vi "Main.vi"() -> ()   [LabVIEW 2015] (continued)
                n1016 = local read "G_max"() -> (w1896:dbl)
                n1017 = local read "G_min"() -> (w1895:dbl)
                n1018 = local read "S_max"() -> (w1894:dbl)
                n1019 = local read "S_min"() -> (w1893:dbl)
                n1020 = Square(x=w1924) -> (x^2=w1922:dbl)
                n1021 = Square(x=w1923) -> (x^2=w1921:dbl)
                n1022 = Add(x=w1922, y=w1921) -> (x+y=w1920:dbl)
                n1023 = Square Root(x=w1920) -> (sqrt(x)=w1919:dbl)
                n1024 = call "DrawROICircle.vi"("old picture"=w1917, "ROI?"=w1912, "Radius (G/S)"=w1911, "Center (G/S)"=w1910, "PicSize"=w1916, "Color"=w1909, "G_max"=w1896, "S_max"=w1894, "G_min"=w1895, "S_min"=w1893) -> ("new picture"=w1915:picture)  [unwired: 9 in]
                n1025 = call "DrawROICircle.vi"("old picture"=w1915, "ROI?"=w1907, "Radius (G/S)"=w1908, "Center (G/S)"=w1898, "PicSize"=w1916, "Color"=w1906, "G_max"=w1896, "S_max"=w1894, "G_min"=w1895, "S_min"=w1893) -> ("new picture"=w1903:picture)  [unwired: 9 in]
                n1026 = call "DrawROICircle.vi"("old picture"=w1903, "ROI?"=w1892, "Radius (G/S)"=w1905, "Center (G/S)"=w1897, "PicSize"=w1916, "Color"=w1904, "G_max"=w1896, "S_max"=w1894, "G_min"=w1895, "S_min"=w1893) -> ("new picture"=w1914:picture)  [unwired: 9 in]
                n1027 = call "DrawROICircle.vi"("old picture"=w1914, "ROI?"=w1902, "Radius (G/S)"=w1901, "Center (G/S)"=w1900, "PicSize"=w1916, "Color"=w1899, "G_max"=w1896, "S_max"=w1894, "G_min"=w1895, "S_min"=w1893) -> ("new picture"=w1913:picture)  [unwired: 9 in]
                n1028 = case shown="\"ROI4\"" w1918 {
                  tunnel: w1919 -> [_ w1928 w1929 w1930 w1931]
                  frame "None" {
                  }
                  frame "ROI1" {
                    "Radius1" <- w1928
                  }
                  frame "ROI2" {
                    "Radius2" <- w1929
                  }
                  frame "ROI3" {
                    "Radius3" <- w1930
                  }
                  frame "ROI4" {
                    "Radius4" <- w1931
                  }
                }
              }
            }
          }
        }
        n1029 = property on="Phasor Plot" class="IntGraph (strict)"(error in=w1816, "PlotImages.Front"=w1817) -> (error out=w1822:errorcluster)  [unwired: 1 in, 1 out]
      }
      event "Phasor Plot": Mouse Up; "ROI1?", "ROI2?", "ROI3?", "ROI4?", "Phasor\nOverlap?", "Refresh Overlap": Value Change {
        n1030 = event-data() -> ()  [unwired: 1 in, 1 out]
        n1031 = local read "ROI Drawing"() -> (w1976:bool)
        n1032 = local read "ROI Select"() -> (w1977:enum16{"None", "ROI1", "ROI2", "ROI3", "ROI4"})
        n1033 = case shown="True" w1976 {
          tunnel: w1977 -> [_ w2002]
          tunnel: w1969 -> [w1999 w2000]
          tunnel: [w1999 w2000] -> w1968
          frame False {
          }
          frame True {
            n1034 = case shown="\"ROI1\"" w2002 {
              frame "None" {
              }
              frame "ROI1" {
                n1035 = local read "Radius1"() -> (w2007:dbl)
                n1036 = Greater Than 0?(x=w2007) -> (x > 0?=w2006:bool)
                n1037 = Select(t=TRUE ("ROI Drawing"), s=w2006, f=FALSE ("ROI Drawing")) -> (s? t:f=w2005:bool)
                n1038 = local write "ROI1?"(w2005) -> ()
              }
              frame "ROI2" {
                n1039 = local read "Radius2"() -> (w2009:dbl)
                n1040 = Greater Than 0?(x=w2009) -> (x > 0?=w2012:bool)
                n1041 = Select(t=TRUE ("ROI Drawing"), s=w2012, f=FALSE ("ROI Drawing")) -> (s? t:f=w2008:bool)
                n1042 = local write "ROI2?"(w2008) -> ()
              }
              frame "ROI3" {
                n1043 = local read "Radius3"() -> (w2015:dbl)
                n1044 = Greater Than 0?(x=w2015) -> (x > 0?=w2016:bool)
                n1045 = Select(t=TRUE ("ROI Drawing"), s=w2016, f=FALSE ("ROI Drawing")) -> (s? t:f=w2014:bool)
                n1046 = local write "ROI3?"(w2014) -> ()
              }
              frame "ROI4" {
                n1047 = local read "Radius4"() -> (w2019:dbl)
                n1048 = Greater Than 0?(x=w2019) -> (x > 0?=w2022:bool)
                n1049 = Select(t=TRUE ("ROI Drawing"), s=w2022, f=FALSE ("ROI Drawing")) -> (s? t:f=w2018:bool)
                n1050 = local write "ROI4?"(w2018) -> ()
              }
            }
            n1051 = local write "ROI Drawing"(FALSE ("ROI Drawing")) -> ()
          }
        }
        n1052 = local read "Radius4"() -> (w1964:dbl)
        n1053 = local read "Center4"() -> (w1961:cluster{dbl, dbl})
        n1054 = local read "Radius2"() -> (w1966:dbl)
        n1055 = local read "Center2"() -> (w1962:cluster{dbl, dbl})
        n1056 = local read "Radius3"() -> (w1965:dbl)
        n1057 = local read "Center3"() -> (w1952:cluster{dbl, dbl})
        n1058 = local read "Radius1"() -> (w1967:dbl)
        n1059 = local read "Center1"() -> (w1963:cluster{dbl, dbl})
        n1060 = local read "PicSize"() -> (w1972:u32)
        n1061 = local read "Color4"() -> (w1957:u32)
        n1062 = local read "Color2"() -> (w1959:u32)
        n1063 = local read "Color3"() -> (w1958:u32)
        n1064 = local read "Color1"() -> (w1960:u32)
        n1065 = local read "ROI4?"() -> (w1942:bool)
        n1066 = local read "ROI3?"() -> (w1943:bool)
        n1067 = local read "ROI1?"() -> (w1945:bool)
        n1068 = local read "ROI2?"() -> (w1944:bool)
        n1069 = Build Array(w1945, w1944, w1943, w1942) -> (w1941:bool[])
        n1070 = Build Array(w1967, w1966, w1965, w1964) -> (w1940:dbl[])
        n1071 = Build Array(w1963, w1962, w1952, w1961) -> (w1939:cluster{dbl, dbl}[])
        n1072 = local read "G_max"() -> (w1951:dbl)
        n1073 = local read "G_min"() -> (w1950:dbl)
        n1074 = local read "S_max"() -> (w1949:dbl)
        n1075 = Build Array(w1960, w1959, w1958, w1957) -> (w1938:u32[])
        n1076 = local read "S_min"() -> (w1948:dbl)
        n1077 = call "Empty Picture"() -> ("empty picture"=w1970:picture)
        n1078 = call "DrawROICircle.vi"("old picture"=w1970, "ROI?"=w1945, "Radius (G/S)"=w1967, "Center (G/S)"=w1963, "PicSize"=w1972, "Color"=w1960, "G_max"=w1951, "S_max"=w1949, "G_min"=w1950, "S_min"=w1948) -> ("new picture"=w1975:picture)  [unwired: 9 in]
        n1079 = call "DrawROICircle.vi"("old picture"=w1975, "ROI?"=w1944, "Radius (G/S)"=w1966, "Center (G/S)"=w1962, "PicSize"=w1972, "Color"=w1959, "G_max"=w1951, "S_max"=w1949, "G_min"=w1950, "S_min"=w1948) -> ("new picture"=w1973:picture)  [unwired: 9 in]
        n1080 = call "DrawROICircle.vi"("old picture"=w1973, "ROI?"=w1943, "Radius (G/S)"=w1965, "Center (G/S)"=w1952, "PicSize"=w1972, "Color"=w1958, "G_max"=w1951, "S_max"=w1949, "G_min"=w1950, "S_min"=w1948) -> ("new picture"=w1974:picture)  [unwired: 9 in]
        n1081 = call "DrawROICircle.vi"("old picture"=w1974, "ROI?"=w1942, "Radius (G/S)"=w1964, "Center (G/S)"=w1961, "PicSize"=w1972, "Color"=w1957, "G_max"=w1951, "S_max"=w1949, "G_min"=w1950, "S_min"=w1948) -> ("new picture"=w1971:picture)  [unwired: 9 in]
        n1082 = local read "Auto Scale?"() -> (w1936:bool)
        n1083 = local read "Max Intensity"() -> (w1935:dbl)
        n1084 = local read "Min Intensity"() -> (w1934:dbl)
        n1085 = control-ref of="Image with Phasors"() -> (w1954:refnum<vi>)
        n1086 = property on="Phasor Plot" class="IntGraph (strict)"(error in=w1968, "PlotImages.Front"=w1971) -> (error out=w1947:errorcluster)  [unwired: 1 in, 1 out]
        n1087 = Bundle(w1941, w1940, w1939, w1938) -> (→"ROI Cluster":T9)  [unwired: 1 in]
        n1088 = local read "V_DC"() -> (w1953:dbl[][])
        n1089 = case shown="True" "Phasor\nOverlap?" {
          tunnel: w1941 -> [_ w1996]
          tunnel: w1940 -> [_ w1995]
          tunnel: w1939 -> [_ w1994]
          tunnel: w1938 -> [_ w1993]
          tunnel: [w1986 w1992] -> w1955
          tunnel: w1954 -> [w1985 w1991]
          tunnel: w1936 -> [w1983 w1990]
          tunnel: w1935 -> [w1982 w1989]
          tunnel: w1934 -> [w1981 w1988]
          tunnel: w1953 -> [w1984 w1987]
          frame False {
            n1090 = call "Array2GrayPic.vi"("Pic Reference"=w1985, "Threshold (min)"=w1981, "Threshold (max)"=w1982, "Auto Scale?"=w1983, "Intensity"=w1984) -> ("Gray Picture"=w1986:picture)  [unwired: 6 in]
          }
          frame True {
            n1091 = local read "G Data"() -> (w1998:dbl[][])
            n1092 = local read "S Data"() -> (w1997:dbl[][])
            n1093 = call "PhasorROI2IMG.vi"("Intensity"=w1987, "Auto Scale?"=w1990, "Threshold (max)"=w1989, "Threshold (min)"=w1988, "G Data"=w1998, "S Data"=w1997, "Pic Reference"=w1991, "ROI? array"=w1996, "Radius array"=w1995, "Center array"=w1994, "Color array"=w1993) -> ("new picture"=w1992:picture)  [unwired: 8 in]
          }
        }
        n1094 = flat-sequence {
          tunnel: [w1980] -> w1946
          tunnel: w1947 -> [w1980]
          frame #0 {
            n1095 = local write "Refresh Overlap"(FALSE ("Fast Scan")) -> ()
          }
        }
        n1096 = local write "Image with Phasors"(w1955) -> ()
      }
      event "Phasor Grids", "G_max", "G_min", "S_max", "S_min", "Phasor Colormap", "Update Phasor": Value Change {
        n1097 = event-data() -> ()  [unwired: 1 in, 1 out]
        n1098 = local read "Phasor Colormap"() -> (w2028:T8)
        n1099 = local read "Max Intensity"() -> (w2026:dbl)
        n1100 = local read "Min Intensity"() -> (w2025:dbl)
        n1101 = local read "Auto Scale?"() -> (w2027:bool)
        n1102 = control-ref of="Phasor Plot"() -> (w2029:refnum<vi>)
        n1103 = local read "Phasor Grids"() -> (w2030:i32)
        n1104 = local read "V_DC"() -> (w2033:dbl[][])
        n1105 = control-ref of="Image with Phasors"() -> (w2042:refnum<vi>)
        n1106 = local read "G Data"() -> (w2032:dbl[][])
        n1107 = local read "S Data"() -> (w2031:dbl[][])
        n1108 = local read "G_max"() -> (w2037:dbl)
        n1109 = local read "G_min"() -> (w2036:dbl)
        n1110 = local read "S_max"() -> (w2035:dbl)
        n1111 = local read "S_min"() -> (w2034:dbl)
        n1112 = call "Array2GrayPic.vi"("Pic Reference"=w2042, "Threshold (min)"=w2025, "Threshold (max)"=w2026, "Auto Scale?"=w2027, "Intensity"=w2033) -> ("Gray Picture"=w2041:picture)  [unwired: 6 in]
        n1113 = call "DrawPhasorPlot.vi"("Intensity"=w2033, "G Data"=w2032, "S Data"=w2031, "Threshold (max)"=w2026, "Threshold (min)"=w2025, "error in"=w2040, "G_max"=w2037, "Auto Scale?"=w2027, "G_min"=w2036, "Phasor Grids"=w2030, "S_max"=w2035, "Reference"=w2029, "S_min"=w2034, "Phasor Colormap"=w2028) -> ("Phasor Plot"=w2038:dbl[][], "error out"=w2039:errorcluster)  [unwired: 4 in]
        n1114 = local write "Image with Phasors"(w2041) -> ()
        n1115 = local write "Phasor Plot"(w2038) -> ()
      }
      event "Load P1": Value Change {
        n1116 = event-data() -> ()  [unwired: 1 in, 1 out]
        n1117 = local read "Measurement Parameters"() -> (w2063:T4)
        n1118 = property on="Composite q1,1" class="Pict"(error in=w2060) -> (error out=w2059:errorcluster, "Draw Area Size"=w2064:T16)  [unwired: 1 in, 1 out]
        n1119 = local read "V_DC"() -> (→"DC,1":dbl[][])
        n1120 = local read "V_IF (pi)"() -> (w2085:dbl[][])
        n1121 = local read "V_IF (0)"() -> (w2084:dbl[][])
        n1122 = local read "V_IF (0.5pi)"() -> (w2083:dbl[][])
        n1123 = local read "V_IF (1.5pi)"() -> (w2082:dbl[][])
        n1124 = Unbundle By Name(w2063) -> ("Pixel Size"=w2062:dbl)
        n1125 = Unbundle By Name(w2064) -> ("Width"=w2065:u32)
        n1126 = To Single Precision Float(number=w2065) -> (single precision float=w2067:sgl)
        n1127 = To Single Precision Float(number=w2062) -> (single precision float=w2066:sgl)
        n1128 = Divide(x=w2067, y=w2066) -> (x/y=w2061:sgl)
        n1129 = Subtract(x=w2085, y=w2084) -> (x-y=w2077:dbl[][])
        n1130 = Subtract(x=w2083, y=w2082) -> (x-y=w2078:dbl[][])
        n1131 = property on="Composite q1,1" class="Pict"(error in=w2059, "ZoomFactor"=w2061) -> (error out=w2055:errorcluster)  [unwired: 1 in, 1 out]
        n1132 = local read "tau_max (s)"() -> (w2057:dbl)
        n1133 = local read "tau_min (s)"() -> (w2056:dbl)
        n1134 = Square(x=w2077) -> (x^2=w2081:dbl[][])
        n1135 = Square(x=w2078) -> (x^2=w2080:dbl[][])
        n1136 = Divide(x=w2077, y=w2078) -> (x/y=w2076:dbl[][])
        n1137 = Add(x=w2081, y=w2080) -> (x+y=w2079:dbl[][])
        n1138 = Inverse Tangent(1:w2076) -> (0:w2073:dbl[][])
        "Angle q1,1" <- w2073
        n1139 = property on="Lifetime q1,1" class="IntGraph (strict)"(error in=w2055, "ZScale.Minimum"=w2056) -> (error out=w2054:errorcluster)  [unwired: 1 in, 1 out]
        n1140 = Square Root(x=w2079) -> (sqrt(x)=w2052:dbl[][])
        "Mag q1,1" <- w2052
        n1141 = Tangent(1:w2073) -> (0:w2072:dbl[][])
        n1142 = Multiply(x=80000000.0, y=6.283185307179586) -> (x*y=w2071:dbl)
        n1143 = local read "Custom Mag?"() -> (w2053:bool)
        n1144 = Divide(x=w2072, y=w2071) -> (x/y=w2070:dbl[][])
        n1145 = property on="Lifetime q1,1" class="IntGraph (strict)"(error in=w2054, "ZScale.Maximum"=w2057) -> (error out=w2051:errorcluster)  [unwired: 1 in, 1 out]
        n1146 = Negate(x=w2070) -> (-x=w2068:dbl[][])
        "Lifetime q1,1" <- w2068
        n1147 = case shown="True" w2053 {
          tunnel: w2052 -> [w2089 _]
          tunnel: [w2088 "q1,1max"] -> w2047
          tunnel: [w2087 "q1,1min"] -> w2048
          frame False {
            n1148 = Array Max & Min(array=w2089) -> (max value=w2088:dbl, min value=w2087:dbl)  [unwired: 2 out]
          }
          frame True {
          }
        }
        n1149 = call "HSVCombIntensityLifetime.vi"("min_intensity"=w2048, "Auto Scale?"=TRUE ("External Bound Intensity Value?"), "max_intensity"=w2047, "lifetime_max (s)"=w2057, "lifetime_min (s)"=w2056, "Lifetime image"=w2068, "Intensity image"=w2052) -> ("HSV to RGB Picture"=→"Composite q1,1":picture)  [unwired: 1 in, 3 out]
        n1150 = property on="Mag q1,1" class="IntGraph (strict)"(error in=w2051, "ZScale.Minimum"=w2048) -> (error out=w2050:errorcluster)  [unwired: 1 in, 1 out]
        n1151 = property on="Mag q1,1" class="IntGraph (strict)"(error in=w2050, "ZScale.Maximum"=w2047) -> (error out=w2049:errorcluster)  [unwired: 1 in, 1 out]
      }
      event "Load P2": Value Change {
        n1152 = event-data() -> ()  [unwired: 1 in, 1 out]
        n1153 = local read "Measurement Parameters"() -> (w2111:T4)
        n1154 = property on="Composite q1,2" class="Pict"(error in=w2110) -> (error out=w2109:errorcluster, "Draw Area Size"=w2108:T16)  [unwired: 1 in, 1 out]
        n1155 = Unbundle By Name(w2111) -> ("Pixel Size"=w2112:dbl)
        n1156 = local read "V_IF (pi)"() -> (w2127:dbl[][])
        n1157 = local read "V_IF (0)"() -> (w2126:dbl[][])
        n1158 = local read "V_IF (0.5pi)"() -> (w2125:dbl[][])
        n1159 = local read "V_IF (1.5pi)"() -> (w2124:dbl[][])
        n1160 = local read "V_DC"() -> (→"DC,2":dbl[][])
        n1161 = Unbundle By Name(w2108) -> ("Width"=w2113:u32)
        n1162 = To Single Precision Float(number=w2113) -> (single precision float=w2115:sgl)
        n1163 = To Single Precision Float(number=w2112) -> (single precision float=w2114:sgl)
        n1164 = Divide(x=w2115, y=w2114) -> (x/y=w2107:sgl)
        n1165 = Subtract(x=w2127, y=w2126) -> (x-y=w2129:dbl[][])
        n1166 = Subtract(x=w2125, y=w2124) -> (x-y=w2130:dbl[][])
        n1167 = property on="Composite q1,2" class="Pict"(error in=w2109, "ZoomFactor"=w2107) -> (error out=w2102:errorcluster)  [unwired: 1 in, 1 out]
        n1168 = local read "tau_max (s)"() -> (w2105:dbl)
        n1169 = local read "tau_min (s)"() -> (w2106:dbl)
        n1170 = Square(x=w2129) -> (x^2=w2133:dbl[][])
        n1171 = Square(x=w2130) -> (x^2=w2132:dbl[][])
        n1172 = Divide(x=w2129, y=w2130) -> (x/y=w2128:dbl[][])
        n1173 = property on="Lifetime q1,2" class="IntGraph (strict)"(error in=w2102, "ZScale.Minimum"=w2106) -> (error out=w2101:errorcluster)  [unwired: 1 in, 1 out]
        n1174 = Add(x=w2133, y=w2132) -> (x+y=w2131:dbl[][])
        n1175 = Inverse Tangent(1:w2128) -> (0:w2095:dbl[][])
        "Angle q1,2" <- w2095
        n1176 = local read "Custom Mag?"() -> (w2104:bool)
        n1177 = property on="Lifetime q1,2" class="IntGraph (strict)"(error in=w2101, "ZScale.Maximum"=w2105) -> (error out=w2100:errorcluster)  [unwired: 1 in, 1 out]
        n1178 = Square Root(x=w2131) -> (sqrt(x)=w2103:dbl[][])
        "Mag q1,2" <- w2103
        n1179 = Tangent(1:w2095) -> (0:w2121:dbl[][])
        n1180 = Multiply(x=80000000.0, y=6.283185307179586) -> (x*y=w2120:dbl)
        n1181 = case shown="True" w2104 {
          tunnel: w2103 -> [w2137 _]
          tunnel: [w2136 "q1,2max"] -> w2097
          tunnel: [w2135 "q1,2min"] -> w2096
          frame False {
            n1182 = Array Max & Min(array=w2137) -> (max value=w2136:dbl, min value=w2135:dbl)  [unwired: 2 out]
          }
          frame True {
          }
        }
        n1183 = Divide(x=w2121, y=w2120) -> (x/y=w2119:dbl[][])
        n1184 = Negate(x=w2119) -> (-x=w2117:dbl[][])
        "Lifetime q1,2" <- w2117
        n1185 = call "HSVCombIntensityLifetime.vi"("min_intensity"=w2096, "Auto Scale?"=TRUE ("External Bound Intensity Value?"), "max_intensity"=w2097, "lifetime_max (s)"=w2105, "lifetime_min (s)"=w2106, "Lifetime image"=w2117, "Intensity image"=w2103) -> ("HSV to RGB Picture"=→"Composite q1,2":picture)  [unwired: 1 in, 3 out]
        n1186 = property on="Mag q1,2" class="IntGraph (strict)"(error in=w2100, "ZScale.Minimum"=w2096) -> (error out=w2099:errorcluster)  [unwired: 1 in, 1 out]
        n1187 = property on="Mag q1,2" class="IntGraph (strict)"(error in=w2099, "ZScale.Maximum"=w2097) -> (error out=w2098:errorcluster)  [unwired: 1 in, 1 out]
      }
      event "Two-Step GSOS": Value Change {
        n1188 = event-data() -> ()  [unwired: 1 in, 1 out]
        n1189 = local read "Measurement Parameters"() -> (w2162:T4)
        n1190 = property on="Composite GSOS" class="Pict"(error in=w2164) -> (error out=w2163:errorcluster, "Draw Area Size"=w2166:T16)  [unwired: 1 in, 1 out]
        n1191 = local read "Mag q1,1"() -> (w2188:dbl[][])
        n1192 = local read "Angle q1,2"() -> (w2149:dbl[][])
        n1193 = local read "Angle q1,1"() -> (w2150:dbl[][])
        n1194 = local read "Mag q1,2"() -> (w2187:dbl[][])
        n1195 = local read "DC,1"() -> (w2145:dbl[][])
        n1196 = local read "DC,2"() -> (w2147:dbl[][])
        n1197 = Unbundle By Name(w2162) -> ("Pixel Size"=w2167:dbl)
        n1198 = Unbundle By Name(w2166) -> ("Width"=w2168:u32)
        n1199 = To Single Precision Float(number=w2168) -> (single precision float=w2170:sgl)
        n1200 = To Single Precision Float(number=w2167) -> (single precision float=w2169:sgl)
        n1201 = Divide(x="P1 Power (au)", y="P2 Power (au)") -> (x/y=w2184:dbl)
        n1202 = Polar To Complex(1:w2149, 2:w2187) -> (0:w2181:cdb[][])
        n1203 = Polar To Complex(1:w2150, 2:w2188) -> (0:w2182:cdb[][])
        n1204 = Square(x=w2184) -> (x^2=w2183:dbl)
        n1205 = Divide(x=w2170, y=w2169) -> (x/y=w2165:sgl)
        n1206 = Negate(x=w2183) -> (-x=w2144:dbl)
        n1207 = property on="Composite GSOS" class="Pict"(error in=w2163, "ZoomFactor"=w2165) -> (error out=w2159:errorcluster)  [unwired: 1 in, 1 out]
        n1208 = To Double Precision Complex(1:w2144) -> (0:w2146:cdb)
        n1209 = local read "tau_max (s)"() -> (w2160:dbl)
        n1210 = local read "tau_min (s)"() -> (w2161:dbl)
        n1211 = Multiply(x=w2181, y=w2146) -> (x*y=w2180:cdb[][])
        n1212 = Multiply(x=w2147, y=w2144) -> (x*y=w2143:dbl[][])
        n1213 = Add(x=w2145, y=w2143) -> (x+y=→"DC,SOS":dbl[][])
        n1214 = Add(x=w2182, y=w2180) -> (x+y=w2179:cdb[][])
        n1215 = property on="Lifetime GSOS" class="IntGraph (strict)"(error in=w2159, "ZScale.Minimum"=w2161) -> (error out=w2158:errorcluster)  [unwired: 1 in, 1 out]
        n1216 = Complex To Polar(r * e^(i*theta)=w2179) -> (r=w2156:dbl[][], theta=w2148:dbl[][])
        "Mag GSOS" <- w2156
        "Angle GSOS" <- w2148
        n1217 = local read "Custom Mag?"() -> (w2157:bool)
        n1218 = property on="Lifetime GSOS" class="IntGraph (strict)"(error in=w2158, "ZScale.Maximum"=w2160) -> (error out=w2155:errorcluster)  [unwired: 1 in, 1 out]
        n1219 = Tangent(1:w2148) -> (0:w2176:dbl[][])
        n1220 = case shown="True" w2157 {
          tunnel: w2156 -> [w2192 _]
          tunnel: [w2191 "qGSmax"] -> w2152
          tunnel: [w2190 "qGSmin"] -> w2151
          frame False {
            n1221 = Array Max & Min(array=w2192) -> (max value=w2191:dbl, min value=w2190:dbl)  [unwired: 2 out]
          }
          frame True {
          }
        }
        n1222 = Multiply(x=80000000.0, y=6.283185307179586) -> (x*y=w2175:dbl)
        n1223 = Divide(x=w2176, y=w2175) -> (x/y=w2174:dbl[][])
        n1224 = Negate(x=w2174) -> (-x=w2172:dbl[][])
        "Lifetime GSOS" <- w2172
        n1225 = call "HSVCombIntensityLifetime.vi"("min_intensity"=w2151, "Auto Scale?"=TRUE ("External Bound Intensity Value?"), "max_intensity"=w2152, "lifetime_max (s)"=w2160, "lifetime_min (s)"=w2161, "Lifetime image"=w2172, "Intensity image"=w2156) -> ("HSV to RGB Picture"=→"Composite GSOS":picture)  [unwired: 1 in, 3 out]
        n1226 = property on="Mag GSOS" class="IntGraph (strict)"(error in=w2155, "ZScale.Minimum"=w2151) -> (error out=w2154:errorcluster)  [unwired: 1 in, 1 out]
        n1227 = property on="Mag GSOS" class="IntGraph (strict)"(error in=w2154, "ZScale.Maximum"=w2152) -> (error out=w2153:errorcluster)  [unwired: 1 in, 1 out]
      }
      event "Export GSOS Images": Value Change {
        n1228 = event-data() -> ()  [unwired: 1 in, 1 out]
        n1229 = local read "Current Directory (2D)?"() -> (w2275:bool)
        n1230 = local read "Mag q1,1"() -> (w2241:dbl[][])
        n1231 = local read "Mag q1,2"() -> (w2240:dbl[][])
        n1232 = local read "Mag GSOS"() -> (w2239:dbl[][])
        n1233 = case shown="True" w2275 {
          tunnel: [w2299 w2300] -> w2274
          frame False {
            n1234 = local read "Save Directory (2D)"() -> (w2299:path)
          }
          frame True {
            n1235 = Current VI's Path() -> (path=w2301:path)
            n1236 = Strip Path(path=w2301) -> (stripped path=w2300:path)  [unwired: 1 out]
          }
        }
        n1237 = local read "Experiment Name (2D)"() -> (w2273:string)
        n1238 = local read "File Name (2D)"() -> (w2248:string)
        n1239 = case shown="True" "Custom Mag?" {
          tunnel: w2241 -> [w2292 _]
          tunnel: [w2291 w2298] -> w2238
          tunnel: [w2290 w2297] -> w2237
          tunnel: [w2288 w2296] -> w2236
          tunnel: [w2289 w2295] -> w2235
          tunnel: [w2287 w2294] -> w2234
          tunnel: [w2286 w2293] -> w2233
          tunnel: w2240 -> [w2285 _]
          tunnel: w2239 -> [w2284 _]
          frame False {
            n1240 = Array Max & Min(array=w2292) -> (max value=w2291:dbl, min value=w2290:dbl)  [unwired: 2 out]
            n1241 = Array Max & Min(array=w2285) -> (max value=w2288:dbl, min value=w2289:dbl)  [unwired: 2 out]
            n1242 = Array Max & Min(array=w2284) -> (max value=w2287:dbl, min value=w2286:dbl)  [unwired: 2 out]
          }
          frame True {
            n1243 = local read "q1,1max"() -> (w2298:dbl)
            n1244 = local read "q1,1min"() -> (w2297:dbl)
            n1245 = local read "q1,2max"() -> (w2296:dbl)
            n1246 = local read "q1,2min"() -> (w2295:dbl)
            n1247 = local read "qGSmax"() -> (w2294:dbl)
            n1248 = local read "qGSmin"() -> (w2293:dbl)
          }
        }
        n1249 = Concatenate Strings(w2273, "_" ("string"), "GSOS" ("string")) -> (w2280:string)
        n1250 = Build Path(base path=w2274, name or relative path=w2280) -> (appended path=w2283:path)
        n1251 = call <vilib>:"Check if File or Folder Exists.vi"("error in (no error)"=w2277, "path"=w2283) -> ("error out"=w2282:errorcluster, "file or folder exists?"=w2272:bool, "dup path"=w2281:path)  [unwired: 7 in]
        n1252 = local read "Lifetime q1,1"() -> (w2258:dbl[][])
        n1253 = case shown="False" w2272 {
          tunnel: w2282 -> [w2305 w2306]
          tunnel: [w2304 w2306] -> w2226
          tunnel: [w2303 w2307] -> w2247
          tunnel: w2281 -> [w2302 w2307]
          frame False {
            n1254 = Create Folder(path (use dialog)=w2302, error in=w2305) -> (created path=w2303:path, error out=w2304:errorcluster)  [unwired: 1 in, 1 out]
          }
          frame True {
          }
        }
        n1255 = local read "Angle q1,1"() -> (w2232:dbl[][])
        n1256 = local read "DC,1"() -> (w2229:dbl[][])
        n1257 = call "HSVCombIntensityLifetime.vi"("min_intensity"=w2237, "Auto Scale?"=FALSE ("External Bound Intensity Value?"), "max_intensity"=w2238, "lifetime_max (s)"="tau_max (s)", "lifetime_min (s)"="tau_min (s)", "Lifetime image"=w2258, "Intensity image"=w2241) -> ("HSV to RGB Picture"=w2260:picture)  [unwired: 1 in, 3 out]
        n1258 = call "Save2RealTIF.vi"("min_value"=w2237, "Specify Range?"=TRUE ("Bound Pixel Value?"), "max_value"=w2238, "Time Stamp?"=FALSE, "File Name Prefix"=w2248, "error in"=w2226, "Identify Name"="q1_Mag" ("string"), "Data 2D Array"=w2241, "Parent Directory"=w2247) -> ("error out"=w2225:errorcluster)  [unwired: 1 in, 1 out]
        n1259 = local read "Angle q1,2"() -> (w2231:dbl[][])
        n1260 = local read "DC,2"() -> (w2228:dbl[][])
        n1261 = local read "Lifetime q1,2"() -> (w2253:dbl[][])
        n1262 = call "HSVCombIntensityLifetime.vi"("min_intensity"=w2235, "Auto Scale?"=FALSE ("External Bound Intensity Value?"), "max_intensity"=w2236, "lifetime_max (s)"="tau_max (s)", "lifetime_min (s)"="tau_min (s)", "Lifetime image"=w2253, "Intensity image"=w2240) -> ("HSV to RGB Picture"=w2256:picture)  [unwired: 1 in, 3 out]
        n1263 = call "Save2RealTIF.vi"("min_value"=w2235, "Specify Range?"=TRUE ("Bound Pixel Value?"), "max_value"=w2236, "Time Stamp?"=FALSE, "File Name Prefix"=w2248, "error in"=w2225, "Identify Name"="q2_Mag" ("string"), "Data 2D Array"=w2240, "Parent Directory"=w2247) -> ("error out"=w2224:errorcluster)  [unwired: 1 in, 1 out]
        n1264 = local read "Angle GSOS"() -> (w2230:dbl[][])
        n1265 = local read "DC,SOS"() -> (w2227:dbl[][])
        n1266 = local read "Lifetime GSOS"() -> (w2246:dbl[][])
        n1267 = call "HSVCombIntensityLifetime.vi"("min_intensity"=w2233, "Auto Scale?"=FALSE ("External Bound Intensity Value?"), "max_intensity"=w2234, "lifetime_max (s)"="tau_max (s)", "lifetime_min (s)"="tau_min (s)", "Lifetime image"=w2246, "Intensity image"=w2239) -> ("HSV to RGB Picture"=w2251:picture)  [unwired: 1 in, 3 out]
        n1268 = call "Save2RealTIF.vi"("min_value"=w2233, "Specify Range?"=TRUE ("Bound Pixel Value?"), "max_value"=w2234, "Time Stamp?"=FALSE, "File Name Prefix"=w2248, "error in"=w2224, "Identify Name"="q2GSOS_Mag" ("string"), "Data 2D Array"=w2239, "Parent Directory"=w2247) -> ("error out"=w2223:errorcluster)  [unwired: 1 in, 1 out]
        n1269 = call "Save2RealTIF.vi"("Specify Range?"=FALSE ("Bound Pixel Value?"), "Time Stamp?"=FALSE, "File Name Prefix"=w2248, "error in"=w2223, "Identify Name"="q1_Angle" ("string"), "Data 2D Array"=w2232, "Parent Directory"=w2247) -> ("error out"=w2222:errorcluster)  [unwired: 3 in, 1 out]
        n1270 = call "Save2RealTIF.vi"("Specify Range?"=FALSE ("Bound Pixel Value?"), "Time Stamp?"=FALSE, "File Name Prefix"=w2248, "error in"=w2222, "Identify Name"="q2_Angle" ("string"), "Data 2D Array"=w2231, "Parent Directory"=w2247) -> ("error out"=w2221:errorcluster)  [unwired: 3 in, 1 out]
        n1271 = call "Save2RealTIF.vi"("Specify Range?"=FALSE ("Bound Pixel Value?"), "Time Stamp?"=FALSE, "File Name Prefix"=w2248, "error in"=w2221, "Identify Name"="q2GSOS_Angle" ("string"), "Data 2D Array"=w2230, "Parent Directory"=w2247) -> ("error out"=w2220:errorcluster)  [unwired: 3 in, 1 out]
        n1272 = call "Save2RealTIF.vi"("Specify Range?"=FALSE ("Bound Pixel Value?"), "Time Stamp?"=FALSE, "File Name Prefix"=w2248, "error in"=w2220, "Identify Name"="DC_1" ("string"), "Data 2D Array"=w2229, "Parent Directory"=w2247) -> ("error out"=w2219:errorcluster)  [unwired: 3 in, 1 out]
        n1273 = call "Save2RealTIF.vi"("Specify Range?"=FALSE ("Bound Pixel Value?"), "Time Stamp?"=FALSE, "File Name Prefix"=w2248, "error in"=w2219, "Identify Name"="DC_2" ("string"), "Data 2D Array"=w2228, "Parent Directory"=w2247) -> ("error out"=w2218:errorcluster)  [unwired: 3 in, 1 out]
        n1274 = call "Save2RealTIF.vi"("Specify Range?"=FALSE ("Bound Pixel Value?"), "Time Stamp?"=FALSE, "File Name Prefix"=w2248, "error in"=w2218, "Identify Name"="DC_SOS" ("string"), "Data 2D Array"=w2227, "Parent Directory"=w2247) -> ("error out"=w2262:errorcluster)  [unwired: 3 in, 1 out]
        n1275 = call "Save2ColorPNG.vi"("Time Stamp?"=FALSE, "File Name Prefix"=w2248, "error in"=w2262, "Identify Name"="q1_Composite" ("string"), "Data Picture"=w2260, "Parent Directory"=w2247) -> ("error out"=w2254:errorcluster)  [unwired: 4 in, 1 out]
        n1276 = call "Save2ColorPNG.vi"("Time Stamp?"=FALSE, "File Name Prefix"=w2248, "error in"=w2254, "Identify Name"="q2_Composite" ("string"), "Data Picture"=w2256, "Parent Directory"=w2247) -> ("error out"=w2249:errorcluster)  [unwired: 4 in, 1 out]
        n1277 = call "Save2ColorPNG.vi"("Time Stamp?"=FALSE, "File Name Prefix"=w2248, "error in"=w2249, "Identify Name"="q2GSOS_Composite" ("string"), "Data Picture"=w2251, "Parent Directory"=w2247) -> ("error out"=w2245:errorcluster)  [unwired: 4 in, 1 out]
      }
      event "tau_max (s)", "tau_min (s)", "q1,1max", "q1,1min", "q1,2max", "q1,2min", "qGSmax", "qGSmin", "Custom Mag?": Value Change {
        n1278 = event-data() -> ()  [unwired: 1 in, 1 out]
        n1279 = local read "tau_max (s)"() -> (w2312:dbl)
        n1280 = local read "tau_min (s)"() -> (w2313:dbl)
        n1281 = property on="Lifetime q1,1" class="IntGraph (strict)"(error in=w2343, "ZScale.Minimum"=w2313) -> (error out=w2342:errorcluster)  [unwired: 1 in, 1 out]
        n1282 = property on="Lifetime q1,1" class="IntGraph (strict)"(error in=w2342, "ZScale.Maximum"=w2312) -> (error out=w2341:errorcluster)  [unwired: 1 in, 1 out]
        n1283 = local read "Lifetime GSOS"() -> (w2311:dbl[][])
        n1284 = local read "Custom Mag?"() -> (w2344:bool)
        n1285 = local read "Lifetime q1,2"() -> (w2320:dbl[][])
        n1286 = local read "Lifetime q1,1"() -> (w2319:dbl[][])
        n1287 = local read "Mag GSOS"() -> (w2314:dbl[][])
        n1288 = local read "Mag q1,2"() -> (w2321:dbl[][])
        n1289 = local read "Mag q1,1"() -> (w2328:dbl[][])
        n1290 = property on="Lifetime q1,2" class="IntGraph (strict)"(error in=w2341, "ZScale.Minimum"=w2313) -> (error out=w2340:errorcluster)  [unwired: 1 in, 1 out]
        n1291 = case shown="True" w2344 {
          tunnel: w2328 -> [w2353 _]
          tunnel: [w2352 w2359] -> w2327
          tunnel: [w2351 w2358] -> w2326
          tunnel: [w2349 w2357] -> w2323
          tunnel: [w2350 w2356] -> w2322
          tunnel: [w2348 w2355] -> w2316
          tunnel: [w2347 w2354] -> w2315
          tunnel: w2321 -> [w2346 _]
          tunnel: w2314 -> [w2345 _]
          frame False {
            n1292 = Array Max & Min(array=w2353) -> (max value=w2352:dbl, min value=w2351:dbl)  [unwired: 2 out]
            n1293 = Array Max & Min(array=w2346) -> (max value=w2349:dbl, min value=w2350:dbl)  [unwired: 2 out]
            n1294 = Array Max & Min(array=w2345) -> (max value=w2348:dbl, min value=w2347:dbl)  [unwired: 2 out]
          }
          frame True {
            n1295 = local read "q1,1max"() -> (w2359:dbl)
            n1296 = local read "q1,1min"() -> (w2358:dbl)
            n1297 = local read "q1,2max"() -> (w2357:dbl)
            n1298 = local read "q1,2min"() -> (w2356:dbl)
            n1299 = local read "qGSmax"() -> (w2355:dbl)
            n1300 = local read "qGSmin"() -> (w2354:dbl)
          }
        }
        n1301 = property on="Lifetime q1,2" class="IntGraph (strict)"(error in=w2340, "ZScale.Maximum"=w2312) -> (error out=w2339:errorcluster)  [unwired: 1 in, 1 out]
        n1302 = property on="Lifetime GSOS" class="IntGraph (strict)"(error in=w2339, "ZScale.Minimum"=w2313) -> (error out=w2338:errorcluster)  [unwired: 1 in, 1 out]
        n1303 = call "HSVCombIntensityLifetime.vi"("min_intensity"=w2326, "Auto Scale?"=TRUE ("External Bound Intensity Value?"), "max_intensity"=w2327, "lifetime_max (s)"=w2312, "lifetime_min (s)"=w2313, "Lifetime image"=w2319, "Intensity image"=w2328) -> ("HSV to RGB Picture"=w2325:picture)  [unwired: 1 in, 3 out]
        n1304 = property on="Lifetime GSOS" class="IntGraph (strict)"(error in=w2338, "ZScale.Maximum"=w2312) -> (error out=w2337:errorcluster)  [unwired: 1 in, 1 out]
        n1305 = call "HSVCombIntensityLifetime.vi"("min_intensity"=w2322, "Auto Scale?"=TRUE ("External Bound Intensity Value?"), "max_intensity"=w2323, "lifetime_max (s)"=w2312, "lifetime_min (s)"=w2313, "Lifetime image"=w2320, "Intensity image"=w2321) -> ("HSV to RGB Picture"=w2318:picture)  [unwired: 1 in, 3 out]
        n1306 = call "HSVCombIntensityLifetime.vi"("min_intensity"=w2315, "Auto Scale?"=TRUE ("External Bound Intensity Value?"), "max_intensity"=w2316, "lifetime_max (s)"=w2312, "lifetime_min (s)"=w2313, "Lifetime image"=w2311, "Intensity image"=w2314) -> ("HSV to RGB Picture"=w2310:picture)  [unwired: 1 in, 3 out]
        n1307 = property on="Mag q1,1" class="IntGraph (strict)"(error in=w2337, "ZScale.Minimum"=w2326) -> (error out=w2336:errorcluster)  [unwired: 1 in, 1 out]
        n1308 = local write "Composite GSOS"(w2310) -> ()
        n1309 = local write "Composite q1,1"(w2325) -> ()
        n1310 = local write "Composite q1,2"(w2318) -> ()
        n1311 = property on="Mag q1,1" class="IntGraph (strict)"(error in=w2336, "ZScale.Maximum"=w2327) -> (error out=w2335:errorcluster)  [unwired: 1 in, 1 out]
        n1312 = property on="Mag q1,2" class="IntGraph (strict)"(error in=w2335, "ZScale.Minimum"=w2322) -> (error out=w2334:errorcluster)  [unwired: 1 in, 1 out]
        n1313 = property on="Mag q1,2" class="IntGraph (strict)"(error in=w2334, "ZScale.Maximum"=w2323) -> (error out=w2333:errorcluster)  [unwired: 1 in, 1 out]
        n1314 = property on="Mag GSOS" class="IntGraph (strict)"(error in=w2333, "ZScale.Minimum"=w2315) -> (error out=w2332:errorcluster)  [unwired: 1 in, 1 out]
        n1315 = property on="Mag GSOS" class="IntGraph (strict)"(error in=w2332, "ZScale.Maximum"=w2316) -> (error out=w2331:errorcluster)  [unwired: 1 in, 1 out]
      }
      event "Save 2D Images": Value Change {
        n1316 = event-data() -> ()  [unwired: 1 in, 1 out]
        n1317 = local read "Current Directory (2D)?"() -> (w2411:bool)
        n1318 = local read "V_DC"() -> (w2367:dbl[][])
        n1319 = local read "Auto Scale?"() -> (w2366:bool)
        n1320 = local read "Current 2D Time-Lapse Meas"() -> (w2369:i32)
        n1321 = case shown="False" w2411 {
          tunnel: ["Save Directory (2D)" w2448] -> w2376
          frame False {
          }
          frame True {
            n1322 = Current VI's Path() -> (path=w2449:path)
            n1323 = Strip Path(path=w2449) -> (stripped path=w2448:path)  [unwired: 1 out]
          }
        }
        n1324 = local read "DC&1w Lifetime (s)"() -> (w2413:dbl[][])
        n1325 = local read "Max Lifetime (s)"() -> (w2414:dbl)
        n1326 = local read "Min Lifetime (s)"() -> (w2415:dbl)
        n1327 = local read "1w Lifetime (s)"() -> (w2412:dbl[][])
        n1328 = local read "V_IF (0.5pi)"() -> (w2395:dbl[][])
        n1329 = local read "V_IF (1.5pi)"() -> (w2393:dbl[][])
        n1330 = local read "V_IF (pi)"() -> (w2394:dbl[][])
        n1331 = local read "V_IF (0)"() -> (w2406:dbl[][])
        n1332 = local read "G Data"() -> (w2374:dbl[][])
        n1333 = local read "S Data"() -> (w2373:dbl[][])
        n1334 = case shown="False" w2366 {
          tunnel: [w2441 w2443] -> w2365
          tunnel: [w2440 w2442] -> w2364
          tunnel: w2367 -> [_ w2444]
          frame False {
            n1335 = local read "Max Intensity"() -> (w2441:dbl)
            n1336 = local read "Min Intensity"() -> (w2440:dbl)
          }
          frame True {
            n1337 = Array Max & Min(array=w2444) -> (max value=w2443:dbl, min value=w2442:dbl)  [unwired: 2 out]
          }
        }
        n1338 = Number To Decimal String(number=w2369) -> (decimal integer string=w2362:string)  [unwired: 1 in]
        n1339 = call "SaveMatrix.vi"("Experiment Name"="Experiment Name (2D)", "Identify Name"="I" ("string"), "Data"=w2367, "matrix_max"=w2365, "matrix_min"=w2364, "error in"=w2392, "File Name"="File Name (2D)", "Index Name"=w2362, "path"=w2376, "Specify Range?"=FALSE ("Bound Pixel Value?"), "Enable?"="Intensity?", "Crop Pixels"="Crop Pixels", "Time Stamp?"="Time Stamp?") -> ("error out"=w2424:errorcluster)  [unwired: 5 in, 1 out]
        n1340 = call "SaveMatrix.vi"("Experiment Name"="Experiment Name (2D)", "Identify Name"="Tau1" ("string"), "Data"=w2412, "error in"=w2424, "File Name"="File Name (2D)", "Index Name"=w2362, "path"=w2376, "Specify Range?"=FALSE ("Bound Pixel Value?"), "Enable?"="1w Lifetime?", "Crop Pixels"="Crop Pixels", "Time Stamp?"="Time Stamp?") -> ("error out"=w2425:errorcluster)  [unwired: 7 in, 1 out]
        n1341 = call "SaveMatrix.vi"("Experiment Name"="Experiment Name (2D)", "Identify Name"="Tau01" ("string"), "Data"=w2413, "error in"=w2425, "File Name"="File Name (2D)", "Index Name"=w2362, "path"=w2376, "Specify Range?"=FALSE ("Bound Pixel Value?"), "Enable?"="DC&1w Lifetime?", "Crop Pixels"="Crop Pixels", "Time Stamp?"="Time Stamp?") -> ("error out"=w2427:errorcluster)  [unwired: 7 in, 1 out]
        n1342 = call "SaveHSVComb.vi"("File Name"="File Name (2D)", "Intensity"=w2367, "intensity_max"=w2365, "intensity_min"=w2364, "Lifetime"=w2412, "lifetime_max (s)"=w2414, "lifetime_min (s)"=w2415, "error in"=w2427, "Experiment Name"="Experiment Name (2D)", "Index Name"=w2362, "Identify Name"="Comp1" ("string"), "Enable?"="1w Composite?", "path"=w2376, "Crop Pixels"="Crop Pixels", "Time Stamp?"="Time Stamp?") -> ("error out"=w2429:errorcluster)  [unwired: 11 in, 1 out]
        n1343 = call "SaveHSVComb.vi"("File Name"="File Name (2D)", "Intensity"=w2367, "intensity_max"=w2365, "intensity_min"=w2364, "Lifetime"=w2413, "lifetime_max (s)"=w2414, "lifetime_min (s)"=w2415, "error in"=w2429, "Experiment Name"="Experiment Name (2D)", "Index Name"=w2362, "Identify Name"="Comp01" ("string"), "Enable?"="DC&1w Composite?", "path"=w2376, "Crop Pixels"="Crop Pixels", "Time Stamp?"="Time Stamp?") -> ("error out"=w2431:errorcluster)  [unwired: 11 in, 1 out]
        n1344 = call "SaveMatrix.vi"("Experiment Name"="Experiment Name (2D)", "Identify Name"="G" ("string"), "Data"=w2374, "error in"=w2431, "File Name"="File Name (2D)", "Index Name"=w2362, "path"=w2376, "Specify Range?"=FALSE ("Bound Pixel Value?"), "Enable?"="G?", "Crop Pixels"="Crop Pixels", "Time Stamp?"="Time Stamp?") -> ("error out"=w2432:errorcluster)  [unwired: 7 in, 1 out]
        n1345 = call "SaveMatrix.vi"("Experiment Name"="Experiment Name (2D)", "Identify Name"="S" ("string"), "Data"=w2373, "error in"=w2432, "File Name"="File Name (2D)", "Index Name"=w2362, "path"=w2376, "Specify Range?"=FALSE ("Bound Pixel Value?"), "Enable?"="S?", "Crop Pixels"="Crop Pixels", "Time Stamp?"="Time Stamp?") -> ("error out"=w2407:errorcluster)  [unwired: 7 in, 1 out]
        n1346 = call "SaveMatrix.vi"("Experiment Name"="Experiment Name (2D)", "Identify Name"="Mix1" ("string"), "Data"=w2406, "error in"=w2407, "File Name"="File Name (2D)", "Index Name"=w2362, "path"=w2376, "Specify Range?"=FALSE ("Bound Pixel Value?"), "Enable?"="4 Mix?", "Crop Pixels"="Crop Pixels", "Time Stamp?"="Time Stamp?") -> ("error out"=w2399:errorcluster)  [unwired: 7 in, 1 out]
        n1347 = call "SaveMatrix.vi"("Experiment Name"="Experiment Name (2D)", "Identify Name"="Mix2" ("string"), "Data"=w2395, "error in"=w2399, "File Name"="File Name (2D)", "Index Name"=w2362, "path"=w2376, "Specify Range?"=FALSE ("Bound Pixel Value?"), "Enable?"="4 Mix?", "Crop Pixels"="Crop Pixels", "Time Stamp?"="Time Stamp?") -> ("error out"=w2398:errorcluster)  [unwired: 7 in, 1 out]
        n1348 = call "SaveMatrix.vi"("Experiment Name"="Experiment Name (2D)", "Identify Name"="Mix3" ("string"), "Data"=w2394, "error in"=w2398, "File Name"="File Name (2D)", "Index Name"=w2362, "path"=w2376, "Specify Range?"=FALSE ("Bound Pixel Value?"), "Enable?"="4 Mix?", "Crop Pixels"="Crop Pixels", "Time Stamp?"="Time Stamp?") -> ("error out"=w2397:errorcluster)  [unwired: 7 in, 1 out]
        n1349 = local read "Phasor Grids"() -> (w2387:i32)
        n1350 = local read "ROI Cluster"() -> (w2379:T9)
        n1351 = local read "G_max"() -> (w2385:dbl)
        n1352 = local read "G_min"() -> (w2384:dbl)
        n1353 = local read "S_max"() -> (w2383:dbl)
        n1354 = local read "S_min"() -> (w2382:dbl)
        n1355 = flat-sequence {
          tunnel: w2380 -> [w2446]
          tunnel: [w2446] -> w2410
          frame #0 {
            n1356 = local write "Save 2D Images"(FALSE ("Save 3D Stacks")) -> ()
          }
        }
        n1357 = call "SaveMatrix.vi"("Experiment Name"="Experiment Name (2D)", "Identify Name"="Mix4" ("string"), "Data"=w2393, "error in"=w2397, "File Name"="File Name (2D)", "Index Name"=w2362, "path"=w2376, "Specify Range?"=FALSE ("Bound Pixel Value?"), "Enable?"="4 Mix?", "Crop Pixels"="Crop Pixels", "Time Stamp?"="Time Stamp?") -> ("error out"=w2391:errorcluster)  [unwired: 7 in, 1 out]
        n1358 = call "SavePhasor.vi"("Intensity"=w2367, "G Data"=w2374, "S Data"=w2373, "Threshold (max)"=w2365, "Threshold (min)"=w2364, "Auto Scale?"=FALSE, "Phasor Grids"=w2387, "error in"=w2391, "G_max"=w2385, "Index Name"=w2362, "G_min"=w2384, "S_max"=w2383, "Enable?"="Phasor?", "S_min"=w2382, "Time Stamp?"="Time Stamp?", "path"=w2376, "Experiment Name"="Experiment Name (2D)", "File Name"="File Name (2D)", "Identify Name"="Phasor" ("string"), "Crop Pixels"="Crop Pixels") -> ("error out"=w2381:errorcluster)  [unwired: 6 in, 1 out]
        n1359 = call "SaveOverlap.vi"("ROI Cluster"=w2379, "Intensity"=w2367, "Auto Scale?"=FALSE, "Threshold (max)"=w2365, "Threshold (min)"=w2364, "G Data"=w2374, "S Data"=w2373, "error in"=w2381, "File Name"="File Name (2D)", "Index Name"=w2362, "Experiment Name"="Experiment Name (2D)", "Time Stamp?"="Time Stamp?", "Identify Name"="Overlap" ("string"), "Enable?"="Overlap?", "path"=w2376, "Crop Pixels"="Crop Pixels") -> ("error out"=w2380:errorcluster)  [unwired: 10 in, 1 out]
      }
      event "Current Directory (2D)?": Value Change {
        n1360 = event-data() -> ()  [unwired: 1 in, 1 out]
        n1361 = case shown="True" "Current Directory (2D)?" {
          frame False {
          }
          frame True {
            n1362 = Current VI's Path() -> (path=w2456:path)
            n1363 = Strip Path(path=w2456) -> (stripped path=w2455:path)  [unwired: 1 out]
            n1364 = local write "Save Directory (2D)"(w2455) -> ()
          }
        }
      }
      event "Shutter": Value Change {
        n1365 = event-data() -> ()  [unwired: 1 in, 1 out]
        n1366 = call "ShutterControl.vi"("error in"=w2461, "Shutter"="Shutter") -> ("error out"=w2460:errorcluster)  [unwired: 8 in, 1 out]
      }
      event "Power Rotate": Value Change {
        n1367 = event-data() -> ()  [unwired: 1 in, 1 out]
        n1368 = call "PowerControl.vi"("error in"=w2468, "Pulses\n(/0.45°)"="Pulses\n(/0.45°)", "Direction"="Direction") -> ("error out"=w2467:errorcluster)  [unwired: 8 in]
      }
      event "Stop": Value Change {
        n1369 = event-data() -> ()  [unwired: 1 in, 1 out]
        n1370 = call "ShutterControl.vi"("error in"=w2478, "Shutter"=FALSE) -> ("error out"=w2477:errorcluster, "Status Indicator"=w2473:bool)  [unwired: 8 in]
        n1371 = local write "Shutter"(w2473) -> ()
        n1372 = local write "Fast Scan Progress"(0.0 ("Fast Scan Progress")) -> ()
        n1373 = local write "Meas Progress"(0.0 ("Fast Scan Progress")) -> ()
        n1374 = local write "Measure"(FALSE ("Fast Scan")) -> ()
        n1375 = local write "Fast Scan"(FALSE ("Fast Scan")) -> ()
      }
      event "X+": Value Change {
        w2491 = "," ("string")
        n1376 = event-data() -> ()  [unwired: 1 in, 1 out]
        n1377 = Number To Decimal String(number="XY Step (um)") -> (decimal integer string=w2490:string)  [unwired: 1 in]
        n1378 = Concatenate Strings("X" ("string"), w2491, w2490, w2491, w2490, "\r", "R" ("string")) -> (w2489:string)
        n1379 = VISA Write(VISA resource name=w2498, write buffer=w2489, error in (no error)=w2497) -> (VISA resource name out=w2496:refnum<visa-resource-name>, error out=w2495:errorcluster)  [unwired: 1 out]
        n1380 = VISA Read(VISA resource name=w2496, byte count=u32 256, error in (no error)=w2495) -> (VISA resource name out=w2483:refnum<visa-resource-name>, error out=w2484:errorcluster)  [unwired: 2 out]
        n1381 = VISA Clear(VISA resource name=w2483, error in (no error)=w2484) -> (VISA resource name out=w2486:refnum<visa-resource-name>, error out=w2485:errorcluster)
      }
      event "X-": Value Change {
        w2509 = "," ("string")
        n1382 = event-data() -> ()  [unwired: 1 in, 1 out]
        n1383 = local read "XY Step (um)"() -> (w2511:u32)
        n1384 = Number To Decimal String(number=w2511) -> (decimal integer string=w2508:string)  [unwired: 1 in]
        n1385 = Concatenate Strings("X" ("string"), w2509, w2508, w2509, w2508, "\r", "L" ("string")) -> (w2505:string)
        n1386 = VISA Write(VISA resource name=w2516, write buffer=w2505, error in (no error)=w2515) -> (VISA resource name out=w2514:refnum<visa-resource-name>, error out=w2513:errorcluster)  [unwired: 1 out]
        n1387 = VISA Read(VISA resource name=w2514, byte count=u32 256, error in (no error)=w2513) -> (VISA resource name out=w2504:refnum<visa-resource-name>, error out=w2501:errorcluster)  [unwired: 2 out]
        n1388 = VISA Clear(VISA resource name=w2504, error in (no error)=w2501) -> (VISA resource name out=w2503:refnum<visa-resource-name>, error out=w2502:errorcluster)
      }
      event "Y+": Value Change {
        w2527 = "," ("string")
        n1389 = event-data() -> ()  [unwired: 1 in, 1 out]
        n1390 = local read "XY Step (um)"() -> (w2529:u32)
        n1391 = Number To Decimal String(number=w2529) -> (decimal integer string=w2526:string)  [unwired: 1 in]
        n1392 = Concatenate Strings("X" ("string"), w2527, w2526, w2527, w2526, "\r", "F" ("string")) -> (w2523:string)
        n1393 = VISA Write(VISA resource name=w2534, write buffer=w2523, error in (no error)=w2533) -> (VISA resource name out=w2531:refnum<visa-resource-name>, error out=w2530:errorcluster)  [unwired: 1 out]
        n1394 = VISA Read(VISA resource name=w2531, byte count=u32 256, error in (no error)=w2530) -> (VISA resource name out=w2519:refnum<visa-resource-name>, error out=w2522:errorcluster)  [unwired: 2 out]
        n1395 = VISA Clear(VISA resource name=w2519, error in (no error)=w2522) -> (VISA resource name out=w2520:refnum<visa-resource-name>, error out=w2521:errorcluster)
      }
      event "Y-": Value Change {
        w2545 = "," ("string")
        n1396 = event-data() -> ()  [unwired: 1 in, 1 out]
        n1397 = local read "XY Step (um)"() -> (w2547:u32)
        n1398 = Number To Decimal String(number=w2547) -> (decimal integer string=w2544:string)  [unwired: 1 in]
        n1399 = Concatenate Strings("X" ("string"), w2545, w2544, w2545, w2544, "\r", "B" ("string")) -> (w2541:string)
        n1400 = VISA Write(VISA resource name=w2552, write buffer=w2541, error in (no error)=w2551) -> (VISA resource name out=w2549:refnum<visa-resource-name>, error out=w2548:errorcluster)  [unwired: 1 out]
        n1401 = VISA Read(VISA resource name=w2549, byte count=u32 256, error in (no error)=w2548) -> (VISA resource name out=w2540:refnum<visa-resource-name>, error out=w2537:errorcluster)  [unwired: 2 out]
        n1402 = VISA Clear(VISA resource name=w2540, error in (no error)=w2537) -> (VISA resource name out=w2539:refnum<visa-resource-name>, error out=w2538:errorcluster)
      }
      event "Z+": Value Change {
        n1403 = event-data() -> ()  [unwired: 1 in, 1 out]
        n1404 = Number To Decimal String(number="Z Step (.1um)") -> (decimal integer string=w2565:string)  [unwired: 1 in]
        n1405 = Concatenate Strings("C" ("string"), "," ("string"), w2565, "\r", "U" ("string")) -> (w2561:string)
        n1406 = VISA Write(VISA resource name=w2554, write buffer=w2561, error in (no error)=w2553) -> (VISA resource name out=w2569:refnum<visa-resource-name>, error out=w2568:errorcluster)  [unwired: 1 out]
        n1407 = VISA Read(VISA resource name=w2569, byte count=u32 256, error in (no error)=w2568) -> (VISA resource name out=w2557:refnum<visa-resource-name>, error out=w2560:errorcluster)  [unwired: 2 out]
        n1408 = VISA Clear(VISA resource name=w2557, error in (no error)=w2560) -> (VISA resource name out=w2558:refnum<visa-resource-name>, error out=w2559:errorcluster)
      }
      event "Z-": Value Change {
        n1409 = event-data() -> ()  [unwired: 1 in, 1 out]
        n1410 = local read "Z Step (.1um)"() -> (w2579:u32)
        n1411 = Number To Decimal String(number=w2579) -> (decimal integer string=w2583:string)  [unwired: 1 in]
        n1412 = Concatenate Strings("C" ("string"), "," ("string"), w2583, "\r", "D" ("string")) -> (w2580:string)
        n1413 = VISA Write(VISA resource name=w2572, write buffer=w2580, error in (no error)=w2571) -> (VISA resource name out=w2587:refnum<visa-resource-name>, error out=w2586:errorcluster)  [unwired: 1 out]
        n1414 = VISA Read(VISA resource name=w2587, byte count=u32 256, error in (no error)=w2586) -> (VISA resource name out=w2575:refnum<visa-resource-name>, error out=w2578:errorcluster)  [unwired: 2 out]
        n1415 = VISA Clear(VISA resource name=w2575, error in (no error)=w2578) -> (VISA resource name out=w2576:refnum<visa-resource-name>, error out=w2577:errorcluster)
      }
      event "XY0": Value Change {
        n1416 = event-data() -> ()  [unwired: 1 in, 1 out]
        n1417 = VISA Write(VISA resource name=w2600, write buffer="G,0,0" ("string"), error in (no error)=w2599) -> (VISA resource name out=w2596:refnum<visa-resource-name>, error out=w2595:errorcluster)  [unwired: 1 out]
        n1418 = VISA Read(VISA resource name=w2596, byte count=u32 256, error in (no error)=w2595) -> (VISA resource name out=w2591:refnum<visa-resource-name>, error out=w2592:errorcluster)  [unwired: 2 out]
        n1419 = VISA Clear(VISA resource name=w2591, error in (no error)=w2592) -> (VISA resource name out=w2594:refnum<visa-resource-name>, error out=w2593:errorcluster)
      }
      event "Z0": Value Change {
        n1420 = event-data() -> ()  [unwired: 1 in, 1 out]
        n1421 = VISA Write(VISA resource name=w2610, write buffer="V,0" ("string"), error in (no error)=w2609) -> (VISA resource name out=w2608:refnum<visa-resource-name>, error out=w2607:errorcluster)  [unwired: 1 out]
        n1422 = VISA Read(VISA resource name=w2608, byte count=u32 256, error in (no error)=w2607) -> (VISA resource name out=w2604:refnum<visa-resource-name>, error out=w2603:errorcluster)  [unwired: 2 out]
        n1423 = VISA Clear(VISA resource name=w2604, error in (no error)=w2603) -> (VISA resource name out=w2605:refnum<visa-resource-name>, error out=w2606:errorcluster)
      }
      event "Go to Any XYZ": Value Change {
        w2626 = "," ("string")
        n1424 = event-data() -> ()  [unwired: 1 in, 1 out]
        n1425 = Number To Decimal String(number="X Goal (um)") -> (decimal integer string=w2628:string)  [unwired: 1 in]
        n1426 = Number To Decimal String(number="Y Goal (um)") -> (decimal integer string=w2625:string)  [unwired: 1 in]
        n1427 = Number To Decimal String(number="Z Goal (.1um)") -> (decimal integer string=w2624:string)  [unwired: 1 in]
        n1428 = Concatenate Strings("G" ("string"), w2626, w2628, w2626, w2625, w2626, w2624) -> (w2627:string)
        n1429 = VISA Write(VISA resource name=w2631, write buffer=w2627, error in (no error)=w2630) -> (VISA resource name out=w2620:refnum<visa-resource-name>, error out=w2619:errorcluster)  [unwired: 1 out]
        n1430 = VISA Read(VISA resource name=w2620, byte count=u32 256, error in (no error)=w2619) -> (VISA resource name out=w2615:refnum<visa-resource-name>, error out=w2618:errorcluster)  [unwired: 2 out]
        n1431 = VISA Clear(VISA resource name=w2615, error in (no error)=w2618) -> (VISA resource name out=w2616:refnum<visa-resource-name>, error out=w2617:errorcluster)
      }
      event "Set Current XY to 0": Value Change {
        n1432 = event-data() -> ()  [unwired: 1 in, 1 out]
        n1433 = VISA Write(VISA resource name=w2640, write buffer="PS,0,0" ("string"), error in (no error)=w2639) -> (VISA resource name out=w2642:refnum<visa-resource-name>, error out=w2641:errorcluster)  [unwired: 1 out]
        n1434 = VISA Read(VISA resource name=w2642, byte count=u32 256, error in (no error)=w2641) -> (VISA resource name out=w2635:refnum<visa-resource-name>, error out=w2638:errorcluster)  [unwired: 2 out]